vi "AllIncluded.vi"   [LabVIEW 2009]
uses:
  <instrlib>/niScope/Controls/niScope vertical coupling.ctl
  round2/Pulse Acquisition Method.ctl
  <instrlib>/niScope/Controls/niScope trigger slope.ctl
  <instrlib>/niScope/Controls/niScope trigger source.ctl
  <instrlib>/niScope/Configure/Trigger/niScope Configure Trigger Edge.vi
  <instrlib>/niScope/Acquire/Fetch/niScope Fetch.vi
types:
  T1 = enum16{"open", "replace", "create", "open or create", "replace or create", "replace or create with confirmation"}
  T2 = typedef "Pulse Acquisition Method.ctl" = enum16{"Initialize Batch Acqusition", "Initialize Monitor Acquisition", "Initialize Reference Acquisition", "Perform Batch Acquisition", "Perform Reference Acquisition", "Terminate Batch Acquisition", "Terminate Monitor Acqusition", "Terminate Reference Acquisition", "Standby"}
  T3 = typedef "niScope trigger source.ctl" = string
  T4 = typedef "niScope trigger slope.ctl" = i32
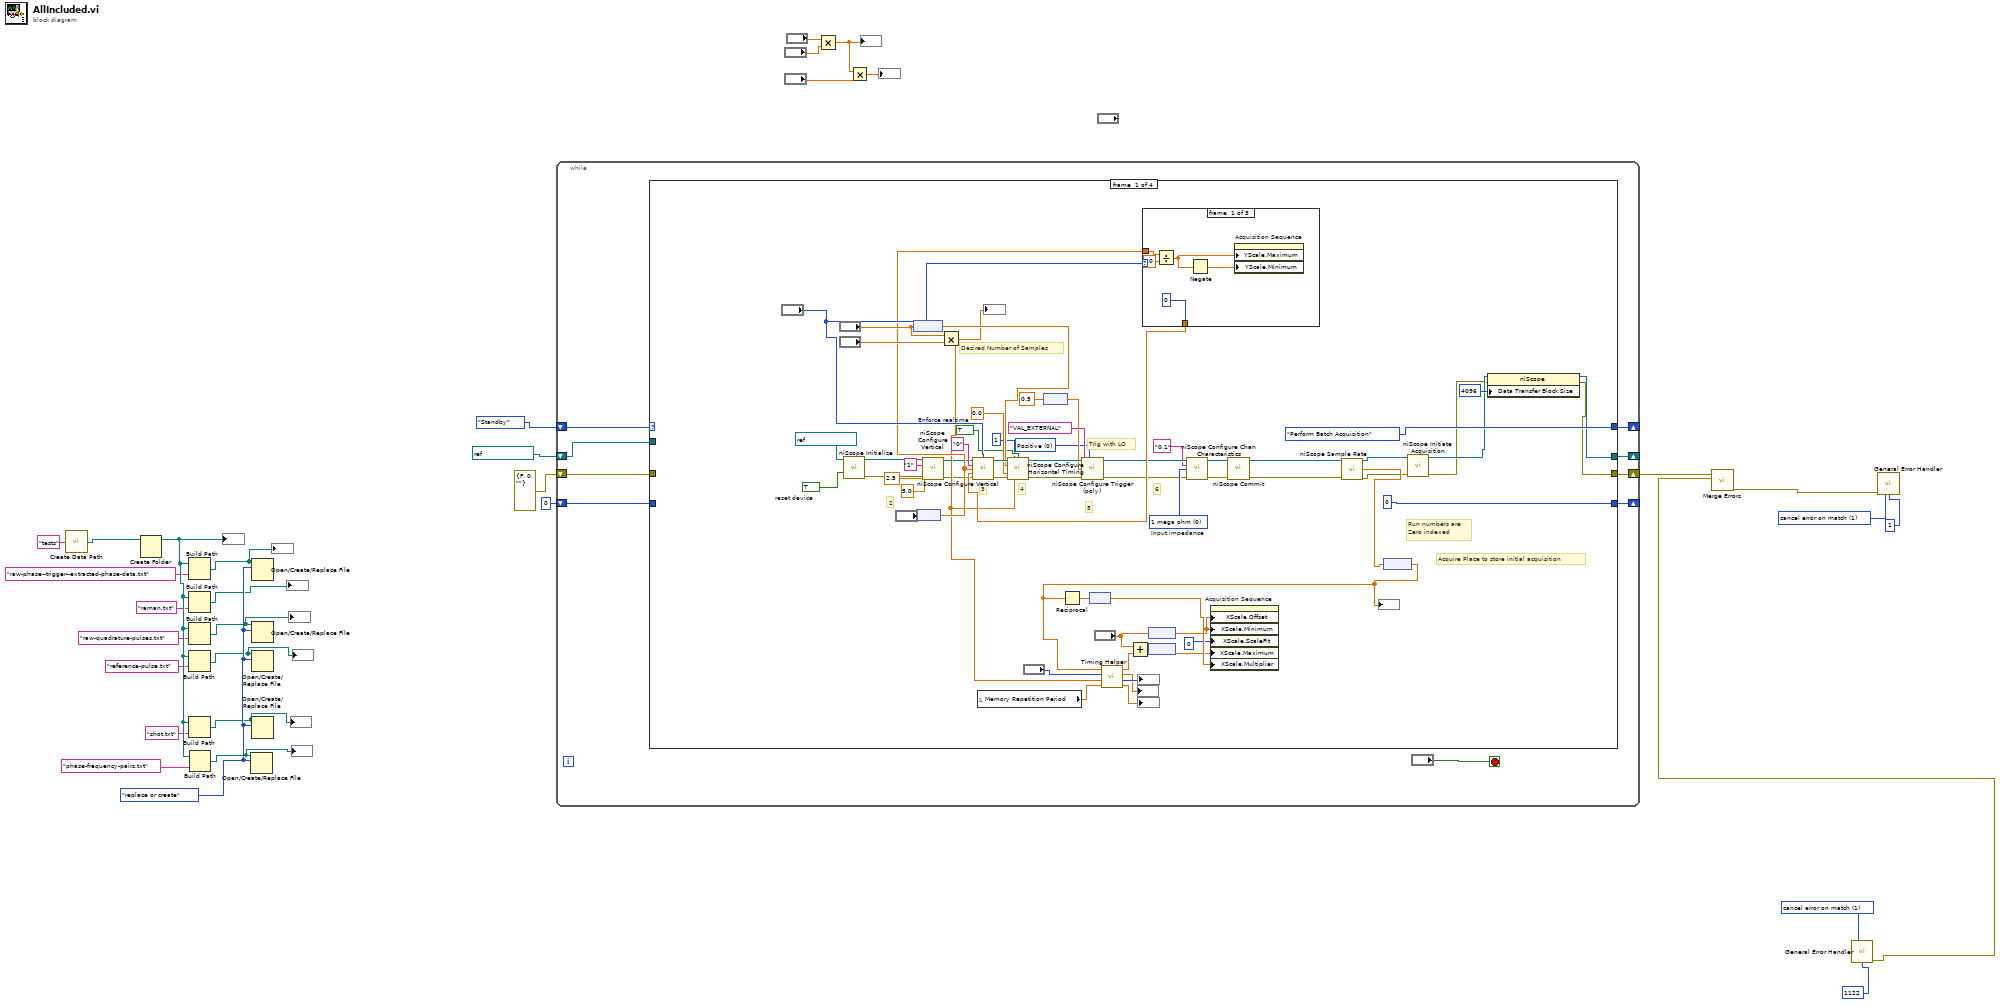
[diagram p0: block diagram]
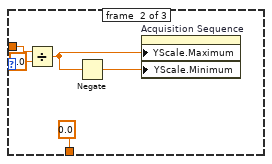
[diagram p2: hidden frame]
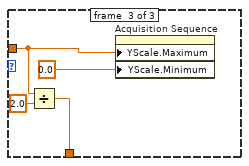
[diagram p3: hidden frame]
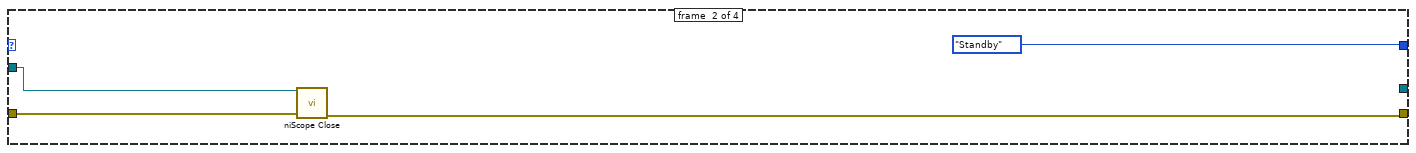
[diagram p4: hidden frame]
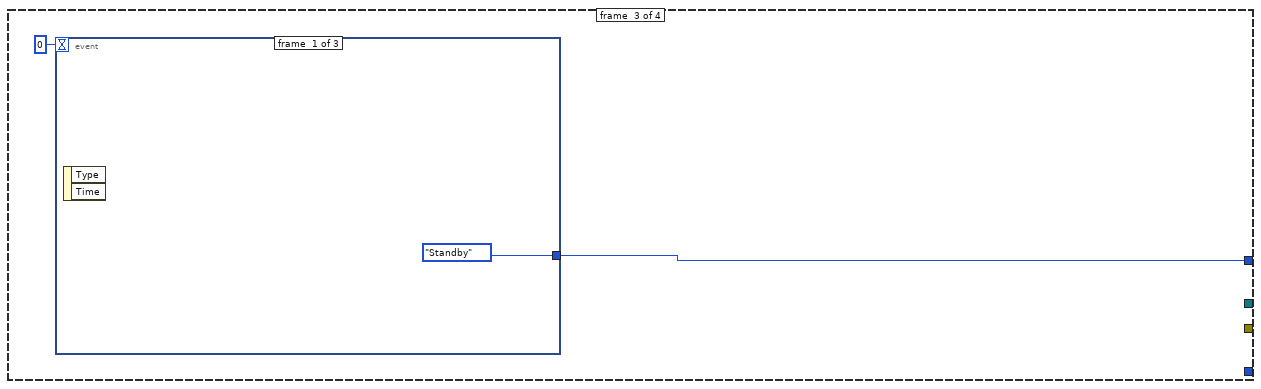
[diagram p5: hidden frame]
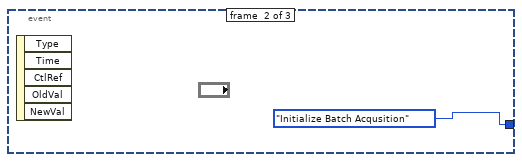
[diagram p6: hidden frame]
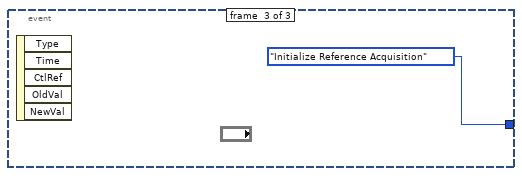
[diagram p7: hidden frame]
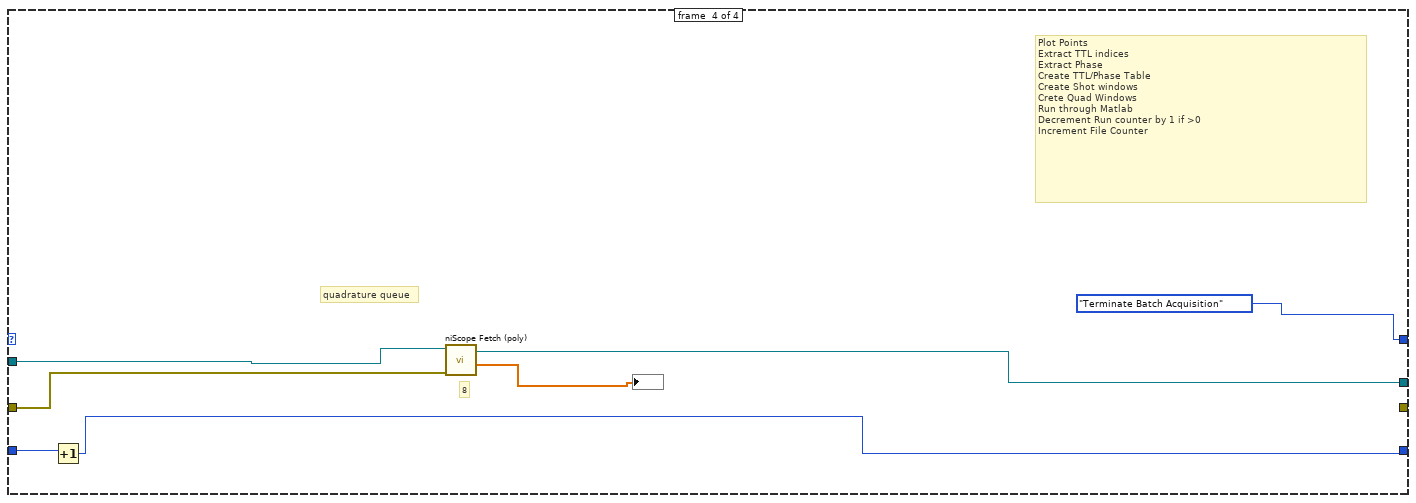
[diagram p8: hidden frame]
diagram:
  w1 = 1 items=["no exception", "cancel error on match", "set error on match"] ("[exception action] (none:0)")
  w5 = 1 items=["no exception", "cancel error on match", "set error on match"] ("[exception action] (none:0)")
  w25 = T1."replace or create" ("operation (0:open)")
  n1 = call "Create Data Path.vi"("Data Directory Name"="tests") -> ("appended path"=w14:path)
  n2 = Create Folder(path (use dialog)=w14) -> (created path=w23:path)  [unwired: 2 in, 2 out]
  "?" <- w23
  n3 = Build Path(base path=w23, name or relative path="raw-phase--trigger--extracted-phase-data.txt") -> (appended path=w16:path)
  "?" <- w16
  n4 = Build Path(base path=w23, name or relative path="raman.txt") -> (appended path=→"?":path)
  n5 = Build Path(base path=w23, name or relative path="raw-quadrature-pulses.txt") -> (appended path=w18:path)
  "?" <- w18
  n6 = Build Path(base path=w23, name or relative path="reference-pulse.txt") -> (appended path=w19:path)
  "?" <- w19
  n7 = Build Path(base path=w23, name or relative path="shot.txt") -> (appended path=w20:path)
  "?" <- w20
  n8 = Build Path(base path=w23, name or relative path="phase-frequency-pairs.txt") -> (appended path=w24:path)
  "?" <- w24
  n9 = Open/Create/Replace File(file path (use dialog)=w24, operation (0:open)=w25) -> ()  [unwired: 4 in, 3 out]
  n10 = Open/Create/Replace File(file path (use dialog)=w16, operation (0:open)=w25) -> ()  [unwired: 4 in, 3 out]
  n11 = Open/Create/Replace File(file path (use dialog)=w18, operation (0:open)=w25) -> ()  [unwired: 4 in, 3 out]
  n12 = Open/Create/Replace File(file path (use dialog)=w19, operation (0:open)=w25) -> ()  [unwired: 4 in, 3 out]
  n13 = Open/Create/Replace File(file path (use dialog)=w20, operation (0:open)=w25) -> ()  [unwired: 4 in, 3 out]
  n14 = while {
    shift-right: [w40] -> _
    shift-left: refnum<k15> "Acquisition" ("instrument handle out") -> [w37]
    shift-right: [w39] -> w26
    shift-left: errorcluster {"status"=FALSE, "code"=0, "source"=""} ("error out") -> [w36]
    shift-right: [w38] -> _
    shift-left: Pulse_Acquisition_Method."Standby" ("Enum") -> [w41]
    shift-right: [w34] -> _
    shift-left: 0 -> [w35]
    stop <- "?" stop-if-true
    n15 = case shown="\"Initialize Batch Acqusition\", Default" w41 {
      tunnel: [w44 _ _ w132] -> w40
      tunnel: [w42 w118 _ _] -> w39
      tunnel: [Pulse_Acquisition_Method."Perform Batch Acquisition" ("Enum") Pulse_Acquisition_Method."Standby" ("Enum") w122 Pulse_Acquisition_Method."Terminate Batch Acquisition" ("Enum")] -> w38
      tunnel: w37 -> [_ w120 _ w130]
      tunnel: w36 -> [_ w119 _ w129]
      tunnel: w35 -> [_ _ _ w131]
      tunnel: [0 _ _ w127] -> w34
      frame #0 {
        w83 = T4 0 items=["Positive", "Negative"] ("trigger slope")
        w79 = TRUE  # Enforce realtime
        w91 = u32 0 items=["1 mega ohm", "75 ohms", "50 ohms"]  # Input impedance
        w102 = TRUE  # reset device
        # "Trig with LO"
        # "Acquire Place to store initial acquisition"
        # "Run numbers are\nZero indexed"
        # "Desired Number of Samples"
        # "6"
        # "5"
        # "4"
        # "3"
        # "2"
        n16 = call <instrlib>:"niScope Initialize.vi"("resource name"=refnum<k15> "Acquisition", "reset device"=w102) -> ("instrument handle"=w55:refnum<k15>, "error out"=w53:errorcluster)  [unwired: 2 in, 10 out]
        n17 = node("?") -> (w80:dbl)
        n18 = node("?") -> (w85:dbl)
        n19 = call <instrlib>:"niScope Configure Vertical.vi"("instrument handle"=w55, "channels"="1", "vertical range"=5.0, "vertical offset"=2.5, "error in"=w53) -> ("instrument handle out"=w54:refnum<k15>, "error out"=w52:errorcluster)  [unwired: 3 in, 6 out]
        n20 = Multiply(x="?", y="?") -> (x*y=w58:dbl)
        "?" <- w58
        n21 = local read "Memory Repetition Period"() -> (w74:dbl[unit])
        n22 = node(dbl[unit] 0.5 ("Trigger level")) -> (w84:dbl)
        n23 = case shown="0, Default" "?" {
          tunnel: w85 -> [w107 w112 w115]
          tunnel: [0 0.0 w113] -> w87
          frame #0 {
            n24 = Divide(x=w107, y=2.0) -> (x/y=w105:dbl)
            n25 = Negate(x=w105) -> (-x=w104:dbl)
            n26 = property on="Acquisition Sequence" class="WFGraph (strict)"("YScale.Maximum"=w105, "YScale.Minimum"=w104) -> ()  [unwired: 2 in, 2 out]
          }
          frame #1 {
            n27 = Divide(x=w112, y=2.0) -> (x/y=w110:dbl)
            n28 = Negate(x=w110) -> (-x=w109:dbl)
            n29 = property on="Acquisition Sequence" class="WFGraph (strict)"("YScale.Maximum"=w110, "YScale.Minimum"=w109) -> ()  [unwired: 2 in, 2 out]
          }
          frame #2 {
            n30 = Divide(x=w115, y=2.0) -> (x/y=w113:dbl)
            n31 = property on="Acquisition Sequence" class="WFGraph (strict)"("YScale.Maximum"=w115, "YScale.Minimum"=0.0 ("Y Scale.Range:Minimum")) -> ()  [unwired: 2 in, 2 out]
          }
        }
        n32 = call <instrlib>:"niScope Configure Vertical.vi"("instrument handle"=w54, "vertical coupling"="?", "channels"="0" ("channel name"), "vertical range"=w85, "vertical offset"=w87, "error in"=w52) -> ("instrument handle out"=w100:refnum<k15>, "error out"=w99:errorcluster)  [unwired: 2 in, 6 out]
        n33 = call <instrlib>:"niScope Configure Horizontal Timing.vi"("instrument handle"=w100, "number of records"=1, "enforce realtime"=w79, "min sample rate"=w80, "reference position"=0.0, "error in"=w99, "min record length"=w58) -> ("instrument handle out"=w98:refnum<k15>, "error out"=w97:errorcluster)  [unwired: 7 out]
        n34 = call-poly <instrlib>:"niScope Configure Trigger (poly).vi"("instrument handle"=w98, "trigger slope"=w83, "trigger source"=T3 "VAL_EXTERNAL", "trigger level"=w84, "error in"=w97) -> ("instrument handle out"=w82:refnum<k15>, "error out"=w81:errorcluster)  [unwired: 3 in, 6 out]
        n35 = node("?") -> (w73:dbl)
        n36 = call <instrlib>:"niScope Configure Chan Characteristics.vi"("instrument handle"=w82, "channels"="0,1", "input impedance"=w91, "error in"=w81) -> ("instrument handle out"=w65:refnum<k15>, "error out"=w64:errorcluster)  [unwired: 1 in, 9 out]
        n37 = call <instrlib>:"niScope Commit.vi"("instrument handle"=w65, "error in"=w64) -> ("instrument handle out"=w63:refnum<k15>, "error out"=w62:errorcluster)  [unwired: 12 in]
        n38 = call <instrlib>:"niScope Sample Rate.vi"("instrument handle"=w63, "error in"=w62) -> ("instrument handle out"=w60:refnum<k15>, "actual sample rate"=w77:dbl, "error out"=w61:errorcluster)  [unwired: 11 out]
        n39 = node(w77) -> (w59:dbl[unit])
        "?" <- w59
        n40 = Reciprocal(x=w59) -> (1/x=w75:dbl[unit])
        n41 = node(w75) -> (w76:dbl)
        n42 = call "Timing Helper.vi"("Repetition Period"=w74, "Number of points per run"=w58, "Number of runs"="?", "Sample rate"=w59) -> ("Total Experiment Time"=→"?":dbl[unit], "Total Number of Datapoints"=→"?":i64, "Total Acquired Time"=→"?":dbl[unit], "Acquisition Time per Run"=w66:dbl[unit])
        n43 = Add(x="?", y=w66) -> (x+y=w70:dbl[unit])
        n44 = node(w70) -> (w72:dbl)
        n45 = property on="Acquisition Sequence" class="WFGraph (strict)"("XScale.Offset"=w73, "XScale.Minimum"=w73, "XScale.ScaleFit"=u8 0 ("X Scale.Scale Fit"), "XScale.Maximum"=w72, "XScale.Multiplier"=w76) -> ()  [unwired: 2 in, 2 out]
        n46 = call <instrlib>:"niScope Initiate Acquisition.vi"("instrument handle"=w60, "error in"=w61) -> ("instrument handle out"=w45:refnum<k15>, "error out"=w43:errorcluster)  [unwired: 12 out]
        n47 = property class="niScope"(reference=w45, error in=w43, "Data Transfer Block Size"=4096) -> (reference out=w44:refnum<k15>, error out=w42:errorcluster)
      }
      frame #1 {
        n48 = call <instrlib>:"niScope Close.vi"("instrument handle"=w120, "error in"=w119) -> ("error out"=w118:errorcluster)  [unwired: 13 out]
      }
      frame #2 {
        n49 = event shown="[2] \"Get Reference Pulse\": Value Change" {
          selector: _ -> [_ _ _]
          dyn-events: _ -> [_ _ _]
          timeout: 0 -> [_ _ _]
          tunnel: [Pulse_Acquisition_Method."Standby" ("Enum") Pulse_Acquisition_Method."Initialize Batch Acqusition" ("Enum") Pulse_Acquisition_Method."Initialize Reference Acquisition" ("Enum")] -> w122
          event #0 {
            n50 = event-data() -> ()  [unwired: 1 in, 2 out]
          }
          event #1 {
            n51 = event-data() -> ()  [unwired: 1 in, 5 out]
          }
          event #2 {
            n52 = event-data() -> ()  [unwired: 1 in, 5 out]
          }
        }
      }
      frame #3 {
        # "Plot Points\nExtract TTL indices\nExtract Phase\nCreate TTL/Phase Table\nCreate Shot windows \nCrete Quad Windows\nRun through Matlab\nDecrement Run counter by 1 if >0\nIncrement File Counter"
        # "quadrature queue"
        # "8"
        n53 = Increment(x=w131) -> (x+1=w127:i32)
        n54 = call-poly <instrlib>:"niScope Fetch (poly).vi"("error in"=w129, "instrument handle"=w130) -> ("wfm"=→"?":dbl[], "instrument handle out"=w132:refnum<k15>)  [unwired: 3 in, 5 out]
      }
    }
  }
  n55 = Multiply(x="?", y="?") -> (x*y=w30:dbl)
  "?" <- w30
  n56 = Multiply(x=w30, y="?") -> (x*y=→"?":dbl)
  n57 = call <vilib>:"General Error Handler.vi"("[exception action] (none:0)"=w1, "[exception code]"=1122 ("[error code] (0)")) -> ("error out"=w3:errorcluster)  [unwired: 9 in, 4 out]
  n58 = call <vilib>:"Merge Errors.vi"("error in 2 (no error)"=w3, "error in 1 (no error)"=w26) -> ("error out"=w6:errorcluster)  [unwired: 2 in, 3 out]
  n59 = call <vilib>:"General Error Handler.vi"("error in (no error)"=w6, "[exception action] (none:0)"=w5, "[exception code]"=1 ("[error code] (0)")) -> ()  [unwired: 8 in, 5 out]
